vi "rs3_SaveOBJ3c.vi"(0 "ppy":sgl=357.0, 1 "fx":sgl=939.0, 2 "RGB image":picture, 3 "MinY":i32=390, 4 "Baseline, mm":dbl=55.0, 5 "fy":sgl=939.0, 7 "ppx":sgl=641.0, 8 "Distortion model":T2(ring), 9 "Save":bool=TRUE, 10 "Obj points and faces":T1(ring), 11 "allowed \ndepth step, mm":dbl=10.0 format="%#_13g", 12 "MinX":i32=670, 13 "MaxY":i32=400, 14 "MaxX":i32=680, 15 "Depth map":dbl[][](array[numeric])=array1280x720[921600 elements], 16 "MinZ":u16=80, 17 "MaxZ":u16=1140, 23 "file path (dialog if empty)":path=path "C:/ProgramData/Obj_and_PNG_Recording/FacePointCloud_3.obj") -> (20 "Density (fill factor)":dbl=1.0 format="%_3g", 21 "subpixel":dbl=0.04032439019607247, 24 "rms error,mm":dbl=0.3624931850372464 format="%0.4f", 25 "rms %":dbl=0.05320098662250997 format="%0.4f", 27 "mean Z Value":dbl=681.3655310743263 format="%0.2f")   [LabVIEW 2017, in "libRealSense3.lvlib"]
uses:
  libRealSense3.lvlib
  <vilib>/Math Plots/3D Math Plots/3D Scatter/3D Scatter XCtrl/3D Scatter.xctl
  <vilib>/Math Plots/3D Math Plots/3D Scatter/3D Scatter Datatype/3D Scatter Datatype.lvclass
  <vilib>/Math Plots/3D Math Plots/3D Scatter/3D Scatter Datatype/Public/Plot Helper (Vector).vi
  <vilib>/Utility/file.llb/Write Delimited Spreadsheet (string).vi
panel:
  out "All vertices":string[][](array[string])
  out "all faces":i32[][](array[numeric])
  out "all vertices":dbl[][](array[numeric])
  out "Face Array":string[][](array[string])
  out "Width":i32=10
  out "Height":i32
  out "new picture":picture
  out "3D point cloud":refnum<class "3D Plot Datatype.lvclass">[](xcontrol)
  # "Save OBJ"
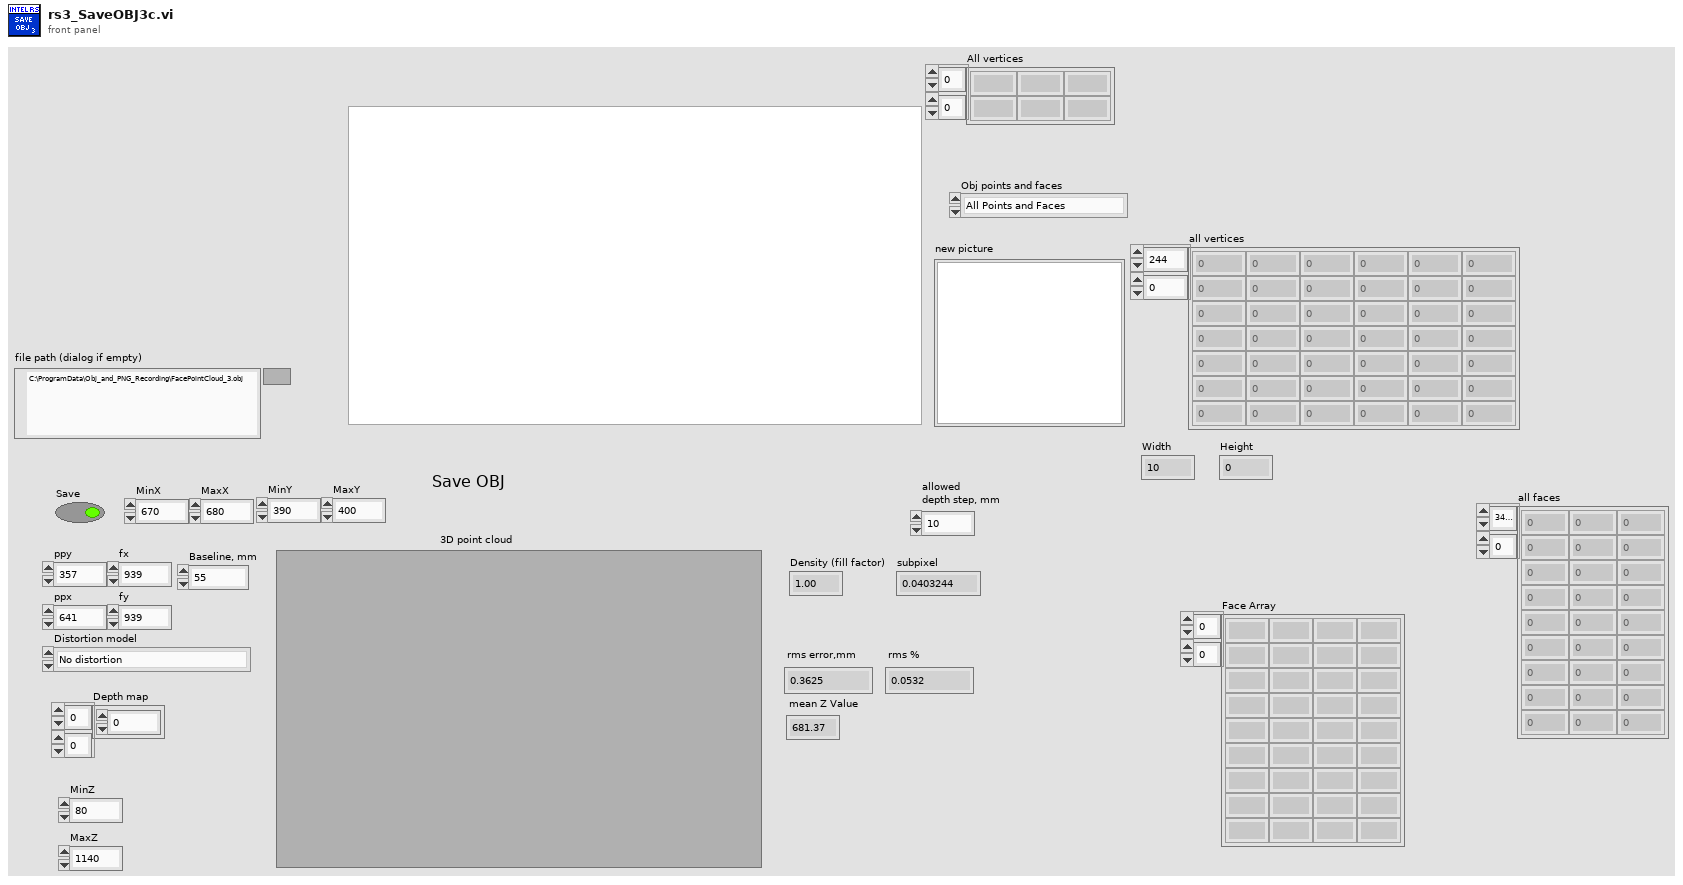
[diagram p1: front panel]
types:
  T1 = enum16{"All Points and Faces", "Only Valid Points", "All point & only Valid Faces", "Only valid Points & Faces "}
  T2 = enum16{"No distortion", "Modified Brown Conrady distortion", "Inverse Brown Conrady distortion", "Distortion Count"}
  T3 = typedef "imagedata.ctl" = cluster{"image type":i32, "image depth":i32, "image":u8[], "mask":u8[], "colors":u32[], "Rectangle":cluster{"left":i16, "top":i16, "right":i16, "bottom":i16}}
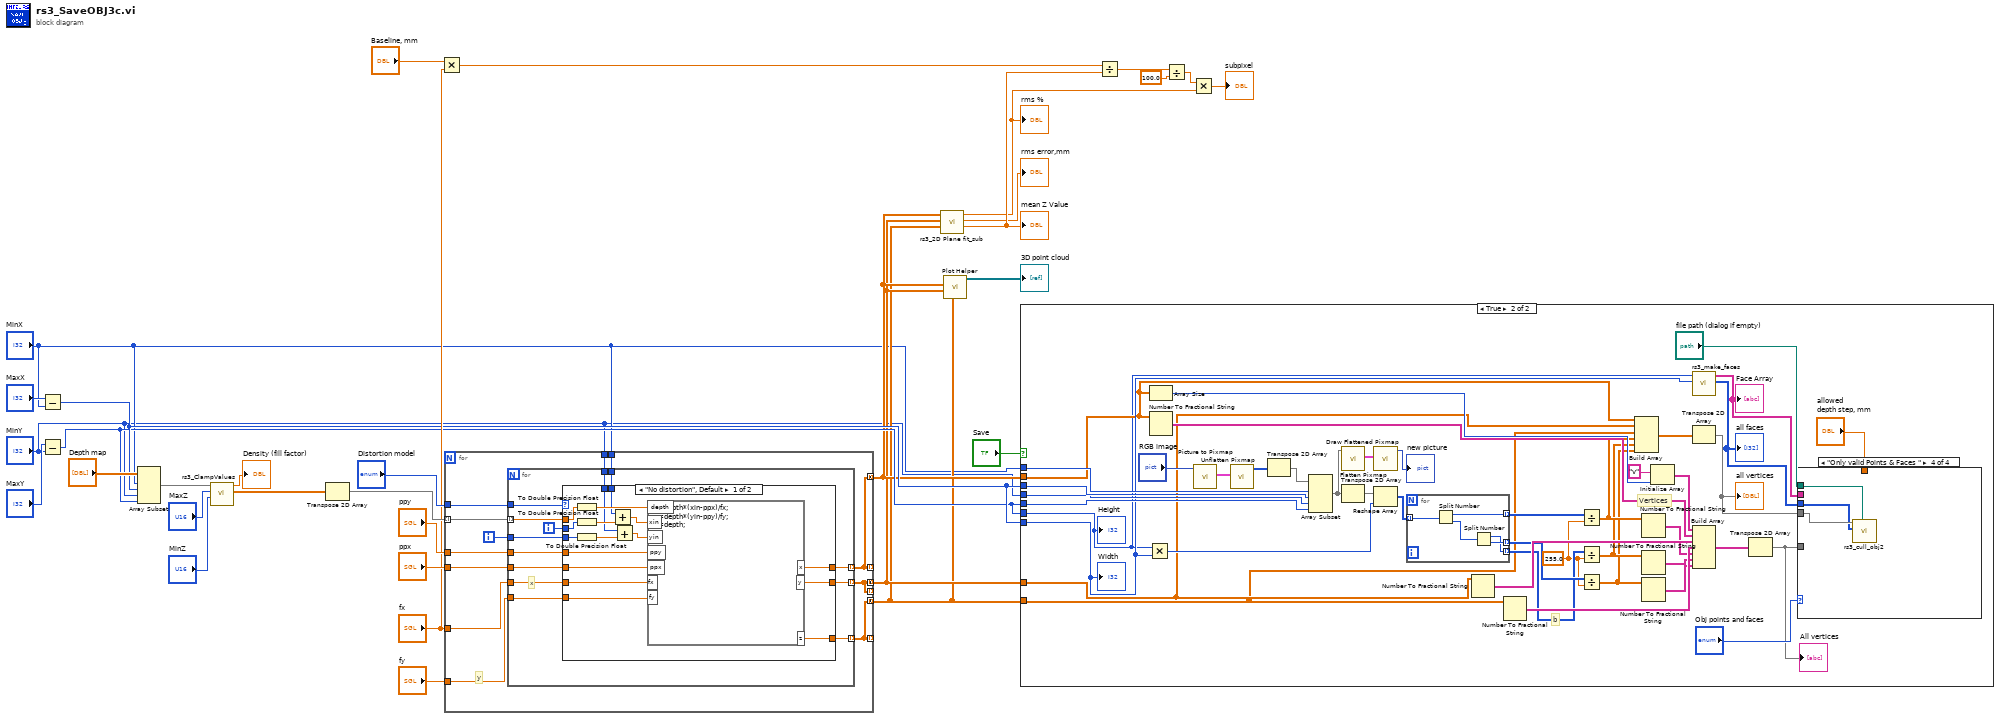
[diagram p0: block diagram]
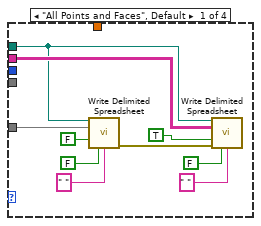
[diagram p3: hidden frame]
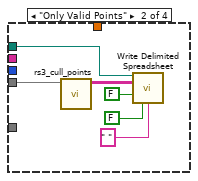
[diagram p4: hidden frame]
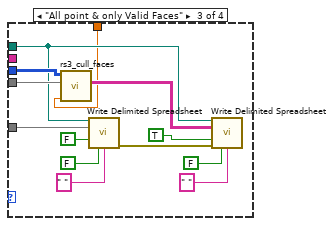
[diagram p5: hidden frame]
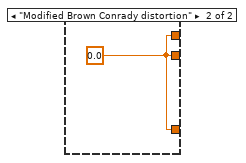
[diagram p6: hidden frame]
diagram:
  n1 = Subtract(x="MaxX", y="MinX") -> (x-y=w7:i32)
  n2 = Subtract(x="MaxY", y="MinY") -> (x-y=w6:i32)
  n3 = Array Subset(array="Depth map", index (row)="MinX", length (row)=w7, index (col)="MinY", length (col)=w6) -> (w10:dbl[][])
  n4 = call "rs3_ClampValues.vi"("MinZ"="MinZ", "MaxZ"="MaxZ", "Depth map"=w10) -> ("Array"=w24:dbl[][], "Density (fill factor)"=→"Density (fill factor)":dbl)  [unwired: 7 in]
  n5 = Transpose 2D Array(2D array=w24) -> (transposed array=w32:dbl[][])
  n6 = Multiply(x="Baseline, mm", y="fx") -> (x*y=w23:dbl)
  n7 = for {
    tunnel: w32 -> [w44] mode=indexing
    tunnel: [w43] -> w5 mode=concatenating
    tunnel: [w42] -> w4 mode=concatenating
    tunnel: [w41] -> w3 mode=concatenating
    tunnel: [w43] -> _ mode=indexing
    tunnel: [w42] -> _ mode=indexing
    tunnel: [w41] -> _ mode=indexing
    tunnel: "ppy" -> [w40]
    tunnel: "ppx" -> [w39]
    tunnel: "fx" -> [w38]
    tunnel: "fy" -> [w37]
    tunnel: "Distortion model" -> [w35]
    tunnel: "MinX" -> [w34]
    tunnel: "MinY" -> [w33]
    i -> [w36]
    # "y"
    n8 = for {
      tunnel: w44 -> [w57] mode=indexing
      tunnel: w36 -> [w56]
      tunnel: [w55] -> w43 mode=indexing
      tunnel: [w54] -> w42 mode=indexing
      tunnel: [w53] -> w41 mode=indexing
      tunnel: w40 -> [w52]
      tunnel: w39 -> [w51]
      tunnel: w38 -> [w50]
      tunnel: w37 -> [w49]
      tunnel: w35 -> [w47]
      tunnel: w34 -> [w46]
      tunnel: w33 -> [w45]
      i -> [w48]
      # "x"
      n9 = case shown="\"No distortion\", Default" w47 {
        tunnel: w57 -> [w70 _]
        tunnel: w48 -> [w69 _]
        tunnel: w56 -> [w68 _]
        tunnel: [w74 w75] -> w55
        tunnel: [w73 w75] -> w54
        tunnel: [w72 w75] -> w53
        tunnel: w52 -> [w67 _]
        tunnel: w51 -> [w66 _]
        tunnel: w50 -> [w65 _]
        tunnel: w49 -> [w64 _]
        tunnel: w46 -> [w62 _]
        tunnel: w45 -> [w59 _]
        frame "No distortion", Default {
          n10 = To Double Precision Float(number=w70) -> (double precision float=w71:dbl)
          n11 = To Double Precision Float(number=w69) -> (double precision float=w63:dbl)
          n12 = To Double Precision Float(number=w68) -> (double precision float=w60:dbl)
          n13 = Add(x=w62, y=w63) -> (x+y=w61:dbl)
          n14 = Add(x=w59, y=w60) -> (x+y=w58:dbl)
          n15 = formula code="x=depth*(xin-ppx)/fx;\ny=depth*(yin-ppy)/fy;\nz=depth;"("ppy"=w67, "ppx"=w66, "fx"=w65, "fy"=w64, "xin"=w61, "yin"=w58, "depth"=w71) -> ("x"=w74:dbl, "y"=w73:dbl, "z"=w72:dbl)
        }
        frame "Modified Brown Conrady distortion" {
          w75 = 0.0 ("x")
        }
      }
    }
  }
  n16 = call "rs3_2D Plane fit_sub.vi"("Z"=w3, "Y"=w4, "X"=w5) -> ("mean Z Value"=w19:dbl, "rms error value"=→"rms error,mm":dbl, "rms %"=w17:dbl)  [unwired: 3 in, 3 out]
  "rms %" <- w17
  "mean Z Value" <- w19
  n17 = call-poly <vilib>:"Plot Helper.vi"("z vector"=w3, "y vector"=w4, "x vector"=w5) -> ("3D Plot lvclass Array out"=→"3D point cloud":refnum<class "3D Plot Datatype.lvclass">[])  [unwired: 3 in, 5 out]
  n18 = case shown="True" "Save" {
    tunnel: w5 -> [_ w91]
    tunnel: w4 -> [_ w90]
    tunnel: w3 -> [_ w89]
    tunnel: "MinX" -> [_ w108]
    tunnel: w7 -> [_ w107]
    tunnel: "MinY" -> [_ w106]
    tunnel: w6 -> [_ w105]
    tunnel: w7 -> [_ w94]
    tunnel: w6 -> [_ w82]
    frame False {
    }
    frame True {
      w99 = 255.0 ("y")
      # "Vertices"
      # "b"
      n19 = Multiply(x=w82, y=w94) -> (x*y=w93:i32)
      n20 = Array Size(array=w91) -> (size(s)=w119:i32)
      n21 = Number To Fractional String(number=w91) -> (F-format string=w116:string[])  [unwired: 3 in]
      n22 = call <vilib>:"Picture to Pixmap.vi"("picture"="RGB image") -> ("image data"=w113:T3)  [unwired: 9 in, 1 out]
      n23 = call <vilib>:"Unflatten Pixmap.vi"("image data"=w113) -> ("24-bit pixmap"=w104:u32[][])  [unwired: 4 in, 6 out]
      n24 = Transpose 2D Array(2D array=w104) -> (transposed array=w103:u32[][])
      n25 = Array Subset(array=w103, index (row)=w108, length (row)=w107, index (col)=w106, length (col)=w105) -> (w96:u32[][])
      n26 = call <vilib>:"Flatten Pixmap.vi"("24-bit pixmap"=w96) -> ("image data"=w98:T3)  [unwired: 10 in]
      n27 = Transpose 2D Array(2D array=w96) -> (transposed array=w92:u32[][])
      n28 = call <vilib>:"Draw Flattened Pixmap.vi"("image data"=w98) -> ("new picture"=→"new picture":picture)  [unwired: 8 in]
      n29 = Reshape Array(w92, w93) -> (w95:u32[])
      n30 = for {
        tunnel: [w155] -> w101 mode=indexing
        tunnel: [w154] -> w100 mode=indexing
        tunnel: [w153] -> w102 mode=indexing
        tunnel: w95 -> [w152] mode=indexing
        n31 = Split Number(x=w152) -> (hi(x)=w153:u16, lo(x)=w156:u16)
        n32 = Split Number(x=w156) -> (hi(x)=w154:u8, lo(x)=w155:u8)
      }
      n33 = Number To Fractional String(number=w90) -> (F-format string=w115:string[])  [unwired: 3 in]
      n34 = Number To Fractional String(number=w89) -> (F-format string=w114:string[])  [unwired: 3 in]
      n35 = Divide(x=w102, y=w99) -> (x/y=w88:dbl[])
      n36 = Divide(x=w100, y=w99) -> (x/y=w87:dbl[])
      n37 = Divide(x=w101, y=w99) -> (x/y=w86:dbl[])
      n38 = Build Array(w91, w90, w89, w88, w87, w86) -> (w85:dbl[][])
      n39 = Number To Fractional String(number=w88) -> (F-format string=w111:string[])  [unwired: 3 in]
      n40 = Number To Fractional String(number=w87) -> (F-format string=w110:string[])  [unwired: 3 in]
      n41 = Number To Fractional String(number=w86) -> (F-format string=w109:string[])  [unwired: 3 in]
      n42 = Initialize Array("v", w119) -> (w117:string[])
      n43 = call "rs3_make_faces.vi"("Width"=w94, "Height"=w82) -> ("all faces"=w80:i32[][], "Face Array"=w81:string[][])  [unwired: 8 in]
      "Face Array" <- w81
      "all faces" <- w80
      n44 = Transpose 2D Array(2D array=w85) -> (transposed array=w84:dbl[][])
      "all vertices" <- w84
      n45 = Build Array(w117, w116, w115, w114, w111, w110, w109) -> (w78:string[][])
      n46 = Transpose 2D Array(2D array=w78) -> (transposed array=w77:string[][])
      "All vertices" <- w77
      n47 = case shown="\"Only valid Points & Faces \"" "Obj points and faces" {
        tunnel: w80 -> [_ _ w147 w150]
        tunnel: w84 -> [_ w131 w148 w151]
        tunnel: "file path (dialog if empty)" -> [w125 w133 w139 w149]
        tunnel: w81 -> [w127 _ _ _]
        tunnel: w77 -> [w124 _ w140 _]
        tunnel: "allowed \ndepth step, mm" -> [_ _ w136 _]
        frame "All Points and Faces", Default {
          n48 = call-poly <vilib>:"Write Delimited Spreadsheet.vi"("file path (dialog if empty)"=w125, "2D data"=w124, "append to file? (new file:F)"=FALSE ("append to file? (F)"), "transpose? (no:F)"=FALSE ("transpose? (F)"), "delimiter (\\t)"=" " ("delimiter (\\t)")) -> ("error out"=w122:errorcluster)  [unwired: 9 in, 1 out]
          n49 = call-poly <vilib>:"Write Delimited Spreadsheet.vi"("file path (dialog if empty)"=w125, "2D data"=w127, "append to file? (new file:F)"=TRUE ("append to file? (F)"), "error in (no error)"=w122, "transpose? (no:F)"=FALSE ("append to file? (F)"), "delimiter (\\t)"=" " ("delimiter (\\t)")) -> ()  [unwired: 8 in, 2 out]
        }
        frame "Only Valid Points" {
          n50 = call "rs3_cull_points.vi"("input vertices"=w131) -> ("Output vertices"=w130:string[][])  [unwired: 8 in, 2 out]
          n51 = call-poly <vilib>:"Write Delimited Spreadsheet.vi"("file path (dialog if empty)"=w133, "2D data"=w130, "append to file? (new file:F)"=FALSE ("append to file? (F)"), "transpose? (no:F)"=FALSE ("transpose? (F)"), "delimiter (\\t)"=" " ("delimiter (\\t)")) -> ()  [unwired: 9 in, 2 out]
        }
        frame "All point & only Valid Faces" {
          n52 = call "rs3_cull_faces.vi"("allowed \ndepth step, mm"=w136, "input vertices"=w148, "Input faces"=w147) -> ("Faces  string"=w144:string[][])  [unwired: 7 in, 1 out]
          n53 = call-poly <vilib>:"Write Delimited Spreadsheet.vi"("file path (dialog if empty)"=w139, "2D data"=w140, "append to file? (new file:F)"=FALSE ("append to file? (F)"), "transpose? (no:F)"=FALSE ("transpose? (F)"), "delimiter (\\t)"=" " ("delimiter (\\t)")) -> ("error out"=w137:errorcluster)  [unwired: 9 in, 1 out]
          n54 = call-poly <vilib>:"Write Delimited Spreadsheet.vi"("file path (dialog if empty)"=w139, "2D data"=w144, "append to file? (new file:F)"=TRUE ("append to file? (F)"), "error in (no error)"=w137, "transpose? (no:F)"=FALSE ("transpose? (F)"), "delimiter (\\t)"=" " ("delimiter (\\t)")) -> ()  [unwired: 8 in, 2 out]
        }
        frame "Only valid Points & Faces " {
          n55 = call "rs3_cull_obj2.vi"("file path (dialog if empty)"=w149, "all faces input"=w150, "vertices"=w151) -> ()  [unwired: 7 in, 2 out]
        }
      }
      "Width" <- w94
      "Height" <- w82
    }
  }
  n56 = Divide(x=w23, y=w19) -> (x/y=w22:dbl)
  n57 = Divide(x=w22, y=100.0) -> (x/y=w21:dbl)
  n58 = Multiply(x=w21, y=w17) -> (x*y=→"subpixel":dbl)
